vi "Controle_Manip_Main_GUI_WorkingBackup_211222.vi"() -> ()   [LabVIEW 2019]
doc: "VI for micro-photoluminescence setup in GH013 to study the emission properties of single nanoemitters in the visible range.\n\nCoded by Mohamed-Raouf Amara"
uses:
  subVIs/TypeDefs/AcqMode.ctl
  C:/Users/manip/Documents/Controle_Manip_2020/Thorlabs.MotionControl.Controls.dll
  Thorlabs.MotionControl.Controls.dll
  C:/Users/manip/Documents/Controle_Manip_2020/Thorlabs.MotionControl.KCube.SolenoidCLI.dll
  Thorlabs.MotionControl.KCube.SolenoidCLI.dll
  C:/Users/manip/Documents/Controle_Manip_2020/Thorlabs.MotionControl.KCube.PiezoCLI.dll
  Thorlabs.MotionControl.KCube.PiezoCLI.dll
  subVIs/Light Field/lightfield-automation-labview/LightField Automation.lvclass
  C:/Program Files/Thorlabs/Scientific Imaging/DCx Camera Support/Develop/DotNet/uc480DotNet.dll
  Program Files/Thorlabs/Scientific Imaging/DCx Camera Support/Develop/DotNet/uc480DotNet.dll
  subVIs/Light Field/lightfield-automation-labview/VIs/TypeDefs/OpticalPortLocation.ctl
  <vilib>/Analysis/baseanly.llb/Mean (DBL).vi
  subVIs/Globals/InstrumentsOn.vi
  subVIs/Globals/InstrumentReferences.vi
  <vilib>/DAQmx/create/channels.llb/DAQmx Create Channel (AO-Voltage-Basic).vi
  subVIs/Attocubes/ANC350_4.2.4_LV16.llb/ANC350v4sub_setFrequency.vi
  subVIs/Attocubes/ANC350_4.2.4_LV16.llb/ANC350v4sub_setAmplitude.vi
  subVIs/Attocubes/ANC350_4.2.4_LV16.llb/ANC350v4sub_getFrequency.vi
  subVIs/Attocubes/ANC350_4.2.4_LV16.llb/ANC350v4sub_getAmplitude.vi
  subVIs/Newport/Newport ESP301/Newport ESP301.lvlib
  <vilib>/Analysis/NI_AALBase.lvlib
panel:
  out "PuissancesPolar":dbl[](array[numeric])
  out "LLTFDevice error out":errorcluster
  out "LLTFDevice Interface":refnum<k7>
  out "LLTF Error":errorcluster
  out "LLTF Reference":refnum<k7>
  in  "xphyspecLib.IXPhySpec":refnum<k7>
  out "PLE 2D ExcWL&Pow":dbl[][](array[numeric])
  out "PLE ExcWL":dbl[](array[numeric])
  out "PLE Norm Int":dbl[][](array[numeric])
  out "PLE Raw Int":i32[][](array[numeric])
  out "PLE IntegInten":dbl[](array[numeric])
  out "PLE ExcPow":dbl[](array[numeric])
  out "Scan Polar AllParams":refnum<vi>[](array[refnum])
  out "Scan PLE AllParams":refnum<vi>[](array[refnum])
  out "Scan PLE Params":refnum<vi>[](array[refnum])
  out "Scan PLE":T1
  out "ExperimentStopped?":bool
  in  "StopPolar":bool
  in  "PausePolar":bool
  out "Elapsed (s)":dbl
  out "Expected (s)":dbl caption="/"
  in  "Stop fPow":bool
  in  "Pause fPow":bool
  in  "MasterStop":bool
  in  "MasterPause":bool
  out "imagefilename":string
  out "Experiment Name With Date":string
  out "FullComment":string
  out "WrittenDatasetName":string
  out "LastDotNum":dbl min=1.0
  out "output cluster":T2
  out "Params Save":T4
  out "Location cluster":T5
  out "Location Parameters":T6
  out "XYPositions":dbl[][](array[numeric])=[[-0.09999999999999998, -0.3], [-0.09999999999999998, -0.19999999999999996], [-0.3, 0.4], [0.20000000000000007, -0.09999999999999998], [-0.5, -0.5], [0.0, 0.20000000000000007], [0.30000000000000004, 0.30000000000000004], [-0.3, -0.5], [-0.5, 0.10000000000000009], [0.0, 0.4], [0.20000000000000007, 0.10000000000000009], [0.30000000000000004, 0.0], [-0.09999999999999998, -0.4], [-0.4, -0.19999999999999996], [-0.5, -0.19999999999999996], [0.4, 0.4], [-0.5, -0.4], [-0.5, -0.3], [-0.19999999999999996, 0.10000000000000009], [-0.19999999999999996, 0.4], [0.4, -0.5], [0.0, 0.10000000000000009], [-0.19999999999999996, 0.0], [0.10000000000000009, 0.30000000000000004], [-0.3, 0.10000000000000009], [0.10000000000000009, -0.3], [0.20000000000000007, -0.4], [-0.09999999999999998, 0.0], [-0.4, -0.5], [-0.5, 0.0], [-0.3, 0.20000000000000007], [-0.5, 0.20000000000000007], [-0.19999999999999996, 0.20000000000000007], [0.5, 0.4], [-0.4, 0.5], [0.5, 0.0], [0.5, 0.20000000000000007], [0.20000000000000007, -0.19999999999999996], [0.10000000000000009, -0.5], [0.4, 0.30000000000000004], [0.10000000000000009, 0.10000000000000009], [-0.4, 0.10000000000000009], [-0.5, 0.30000000000000004], [0.30000000000000004, -0.19999999999999996], [-0.09999999999999998, -0.5], [0.10000000000000009, -0.4], [0.20000000000000007, 0.5], [-0.3, -0.3], [0.4, 0.5], [0.30000000000000004, 0.5], [0.5, -0.3], [-0.09999999999999998, 0.30000000000000004], [0.10000000000000009, 0.20000000000000007], [0.5, 0.10000000000000009], [0.20000000000000007, 0.20000000000000007], [0.5, -0.5], [0.0, -0.5], [0.10000000000000009, 0.0], [0.10000000000000009, -0.19999999999999996], [-0.3, -0.19999999999999996], [-0.4, -0.09999999999999998], [0.20000000000000007, 0.30000000000000004], [0.20000000000000007, -0.5], [-0.3, 0.5], [0.4, 0.10000000000000009], [-0.3, -0.09999999999999998], [0.30000000000000004, -0.4], [0.30000000000000004, 0.10000000000000009], [0.30000000000000004, -0.3], [-0.4, 0.4], [0.5, -0.4], [-0.19999999999999996, -0.19999999999999996], [0.0, -0.19999999999999996], [0.4, 0.20000000000000007], [0.0, 0.0], [0.30000000000000004, 0.20000000000000007], [-0.09999999999999998, 0.5], [-0.3, -0.4], [0.4, -0.3], [0.0, 0.30000000000000004], [0.30000000000000004, 0.4], [0.0, -0.4], [-0.4, 0.30000000000000004], [0.20000000000000007, 0.4], [-0.5, 0.5], [-0.4, -0.4], [0.30000000000000004, -0.5], [0.10000000000000009, 0.4], [-0.09999999999999998, 0.10000000000000009], [0.10000000000000009, 0.5], [-0.4, -0.3], [0.5, -0.09999999999999998], [-0.5, -0.09999999999999998], [0.0, -0.09999999999999998], [-0.19999999999999996, -0.5], [0.4, 0.0], [0.0, -0.3], [-0.19999999999999996, 0.5], [0.5, -0.19999999999999996], [-0.09999999999999998, 0.20000000000000007], [-0.19999999999999996, -0.09999999999999998], [0.20000000000000007, 0.0], [-0.19999999999999996, 0.30000000000000004], [-0.19999999999999996, -0.3], [-0.5, 0.4], [0.10000000000000009, -0.09999999999999998], [-0.19999999999999996, -0.4], [-0.09999999999999998, 0.4], [0.30000000000000004, -0.09999999999999998], [-0.09999999999999998, -0.09999999999999998], [0.20000000000000007, -0.3], [-0.4, 0.20000000000000007], [0.4, -0.4], [-0.3, 0.30000000000000004], [0.5, 0.5], [0.4, -0.19999999999999996], [-0.3, 0.0], [0.0, 0.5], [0.5, 0.30000000000000004], [0.4, -0.09999999999999998], [-0.4, 0.0]]
  in  "DotNum":dbl=1.0 min=1.0
  out "Array fPow Pow":dbl[](array[numeric])
  out "Array fPow":i32[][](array[numeric])
  out "Scan XY Map Exp Params SubVI":T7
  out "Scan XY Map Exp Params SubVI Mod":T8
  out "Scan XY Map References":T9
  in  "Display Mode":u16(ring) items=["Sum", "Max", "Sum/s", "Max/s", "Efficiency"]
  out "BackgroundSpec":dbl[](array[numeric])
  out "Cnts":dbl caption="cnts" format="%_3p"
  out "XYPos Indices":i32[][](array[numeric])
  out "best fit parameters":dbl[](array[numeric])
  out "Image":dbl[][][](array[numeric])
  out "Data PL Custom Diode Spectrum":dbl[](array[numeric])
  out "Out Position [µm | m°]":dbl
  in  "Reset origins":bool
  in  "Delay Line Position (mm)":dbl caption="Delay line position (mm)"
  out "PD Data 2D 2":dbl[][](array[numeric])
  out "PH_Settings_Params":T10={"SyncDiv"=1, "DeviceIndex"=0, "CFD0 level"=50, "CFD0 zero X"=10, "CFD1 level"=50, "CFD1 zero X"=10, "Range No."=0, "StopOnOverflow"=FALSE, "AcqTime (ms)"=0.0} {"Range No." min=0 max=5 step=1; "CFD1 zero X" min=0 max=40 step=1; "CFD1 level" min=0 max=400 step=1; "CFD0 zero X" min=-1300 max=400 step=10; "CFD0 level" min=-1300 max=400 step=10; "SyncDiv" min=1 max=8 step=1}
  out "PH_Init_Data":T11
  out "NewVal":bool
  out "Scan XY Map Handles":T12
  out "Constrast Handles":T13
  out "Contrast References":T14
  in  "Acquire MyPol":bool
  out "Polar Params SubVIv2":T15
  out "Test Handles Polar":T16
  out "Scan Polarisation References":T17
  in  "Att Stop Wobble":bool
  out "Scan Main Progess Bar":u8(slide) scale=0.0..100.0
  out "XYMap Data":i32[][](array[numeric])
  out "PD Data":dbl[](array[numeric])
  out "DDE":refnum<visa-resource-name> caption="resource name"
  in  "Acquire Spectrum Custom":bool
  in  "Stop Spectrum Customm":bool
  out "Scan Spectrum Cust Exp Params":T18
  in  "Experimental parameters tab":T19(tab)
  in  "Save PLE":bool
  in  "Acquire PLE":bool
  in  "PLE Step (nm)":dbl=0.1 caption="Step (nm)" min=0.01 max=100.0 step=0.05
  in  "PLE End (nm)":dbl=500.0 caption="End (nm)" min=300.0 max=1200.0
  in  "PLE Start (nm)":dbl=400.0 caption="Start (nm)" min=300.0 max=1200.0
  out "Background taken?":bool
  in  "Save Custom Diode Spectrum":bool
  in  "Acquire Custom Diode Spectrum":bool
  in  "N Step Power  Diode Current (A)":i32=20 caption="N Steps" min=2 step=1
  in  "End Power  Diod Current (A)":dbl=0.04 caption="End (A)" min=0.02 max=0.0605
  in  "Start Power Diod Current (A)":dbl=0.02 caption="Start (A)" min=0.02 max=0.0605
  in  "Mono2 Wavelength (nm)":dbl=300.0 caption="Wavelength (nm)" min=300.0 max=1000.0 step=0.1
  in  "Mono2 Motor Pos":dbl caption="Motor Pos"
  out "Mono2 On":bool caption="Motor On?"
  in  "CCD ROI":T20(ring) caption="ROI"
  in  "Spectrum Step Wavelength (nm)":dbl=0.25 caption="Step (nm)" min=-100.0 max=100.0 step=0.05
  in  "Spectrum End Wavelength (nm)":dbl=350.0 caption="End (nm)" min=350.0 max=900.0
  in  "Spectrum Start Wavelength (nm)":dbl=350.0 caption="Start (nm)" min=350.0 max=900.0
  in  "Accumulations":dbl=1.0 caption="Acc." min=1.0 step=1.0
  in  "Background substract":enum16{"None", "Shutter"}(ring) caption="Bkg substract"
  in  "Exit mirror":u16(ring)=4 caption="ExitPort :" items=["CCD"=4, "APD"=5]
  in  "Center Wavelength (nm)":dbl=448.9 caption="Center WL :" min=0.0 max=2000.0 step=0.01
  in  "Exposure Time (ms)":dbl=500.0 caption="Exposure :" min=1.0 max=360000.0 step=1.0
  in  "Grating":string(combo)="[h-vis,2400][0][0]" caption="Grating :"
  in  "Spectrum Custom Mode":u16(ring)=1 caption="Detector" items=["PD 1", "APD 1", "APD 2", "APD 1+2", "PD 2"]
  in  "Stop Spectrum Custom":bool
  in  "Save fPow":bool
  in  "Acquire fPow":bool
  in  "HR mode":u16(ring)=1 caption="Which HR?" items=["Excitation"=2, "Detection"=1]
  out "PLE # Pts":dbl=1001.0
  in  "Add location":bool
  in  "Acquire XY Map":bool
  in  "Pause XY Map":bool
  in  "Stop XY Map":bool
  out "Scan X Readout (V)":dbl caption="X Readout" min=-10.0 max=10.0 format="%#.3g"
  out "Scan Y Readout (V)":dbl caption="Y Readout" min=-10.0 max=10.0 format="%#.3g"
  in  "Scan Y Tot. Length":dbl=6.0 caption="Y Length" min=0.0 max=20.0 step=0.5
  in  "Scan X Tot. Length (V)":dbl=6.0 caption="X Length (V)" min=0.0 max=20.0 step=0.5
  out "Scan Y Num. Pts":dbl=121.0 caption="Y # Pts"
  out "Scan X Num. Pts":dbl=121.0 caption="X # Pts"
  in  "Scan Y Res. (V)":dbl=0.05 caption="Res. Y (V)" min=0.0 max=5.0 step=0.05
  in  "Scan X Res. (V)":dbl=0.05 caption="Res. X (V)" min=0.0 max=5.0 step=0.05
  in  "Scan Y Center (V)":dbl caption="Y Center (V)"
  in  "Scan X Center (V)":dbl caption="X Center (V)"
  in  "FSM Home":bool
  in  "FSM Right":bool
  in  "FSM Left":bool
  in  "FSM Down":bool
  in  "FSM Up":bool
  in  "FSM X Axis Pos":dbl caption="Target X" min=-10.0 max=10.0 format="%#.3g"
  in  "FSM Y Axis Pos":dbl caption="Target Y" min=-10.0 max=10.0 format="%#.3f"
  in  "FSM Axis Step":dbl=0.1 caption="Step"
  in  "Save XY Map":bool
  in  "Scanning Mode":T21(ring) caption="Mode"
  in  "Scan Fast Axis":enum16{"Y", "X"}(ring)=enum."X" caption="Fast Axis"
  in  "ZDummyCluster MHILS 3":cluster{"Stop":bool}
  in  "Map Marker X Pos":i8=1 min=1 max=50 step=1
  in  "Map Marker Y Pos":i8=1 min=1 max=50
  in  "Pol in path?":bool
  out "RotStage Det Angle Readout (°)":dbl=2.0 caption="Readout (°)" min=-3600.0 max=125.0 format="%#_4g"
  out "RotStage Exc Angle Readout (°)":dbl=2.0 caption="Readout (°)" min=-360.0 max=360.0 format="%#_4g"
  in  "Acquire Polarisation":bool
  in  "RotStage Det Angle Step (°)":dbl=10.0 caption="Step (°)"
  in  "RotStage Exc Angle Step (°)":dbl=10.0 caption="Step (°)"
  in  "RotStage Det Jog Forward":bool
  in  "RotStage Exc Jog Forward":bool
  in  "RotStage Det Jog Backward":bool
  in  "RotStage Det Home":bool caption="Home"
  in  "RotStage Exc Home":bool caption="Home"
  in  "RotStage Det Angle (°)":dbl caption="Target (°)" min=0.0 max=3600.0 format="%#_4g"
  in  "RotStage Exc Angle (°)":dbl caption="Target (°)" min=0.0 max=3600.0 format="%#_4g"
  in  "RotStage Exc Jog Backward":bool
  in  "Polar Start Angle (°)":dbl caption="Start angle (°)" min=-360.0 max=360.0 step=10.0
  in  "Polar End Angle (°)":dbl=360.0 caption="End Angle (°)" min=0.0 max=360.0 step=10.0
  in  "Polar Step Angle (°)":dbl=10.0 caption="Step Angle (°)" min=0.01 max=360.0
  in  "Polar mode":u16(ring)=3 caption="Rotate HWP" items=["Excitation"=3, "Detection"=2]
  in  "Save Polarisation":bool
  in  "RotStage Det Velocity (°/s)":dbl=2.0 caption="Velocity (°/s)" min=0.0 max=20.0 step=1.0
  in  "RotStage Exc Velocity (°/s)":dbl=2.0 caption="Velocity (°/s)" min=0.0 max=20.0 step=1.0
  in  "Motor RotStage Exc On?":bool
  in  "Motor RotStage Det On?":bool
  in  "ZDummyCluster MHILS 2":cluster{"Stop":bool}
  out "Scan Michelson Progess Bar":u8(slide) scale=0.0..100.0
  in  "Stop Michelson":bool
  in  "Pause Michelson":bool
  in  "Save Michelson":bool
  in  "Acquire Michelson":bool
  in  "Stop Contrast":bool
  in  "Pause Contrast":bool
  in  "Save Contrast":bool
  in  "Newport PZA12 Stage Position (usteps)":dbl caption="Target (ustp)" min=-8.0 max=392.0
  in  "LinTFine Motor On?":bool caption="Motor on?"
  in  "Acquire Contrast":bool
  in  "LinTFines Step Pos (usteps)":dbl=1.0 caption="Step pos (usteps)" min=1.0 max=100.0 step=1.0
  in  "LinTFine End Pos (usteps)":dbl=10.0 caption="End pos (usteps)" min=-1000000.0 max=1000000.0 step=1.0
  in  "LinTFine Start Pos (usteps)":dbl caption="Start pos (usteps)" min=-1000000.0 max=1000000.0 step=1.0
  in  "PZC Speed (usteps/s)":u16(ring) caption="Velocity (ustp/s)" items=["0", "3.2", "16", "80", "400", "2000", "10000", "48000"]
  in  "PZC Jog Forward":bool
  in  "PZC Jog Backward":bool
  in  "PZC Home":bool caption="Home"
  out "PZC Position Readout (usteps)":dbl caption="Readout (ustp)" min=-8.0 max=392.0
  out "Newport Linear Translation Stage Position Readout (mm)":dbl caption="Readout (mm)" min=-8.0 max=392.0 format="%#_7g"
  in  "Newport Linear Translation Stage Step (mm)":dbl=5.0 caption="Step (mm)"
  in  "Newport Linear Translation Stage Position (mm)":dbl caption="Target (mm)" min=-125.0 max=125.0
  out "Scan Linear Stage Progess Bar":u8(slide) scale=0.0..100.0
  in  "Newport Linear Translation Stage Home":bool caption="Home"
  in  "Newport Linear Translation Stage Jog Forward":bool
  in  "Newport Linear Translation Stage Jog Backward":bool
  in  "Newport Linear Translation Stage Velocity (mm/s)":dbl=1.0 caption="Velocity (mm/s)" min=0.0 max=100.0 step=1.0
  in  "LinT Step Pos (mm)":dbl=10.0 caption="Step pos (mm)" min=-50.0 max=50.0 step=0.001
  in  "LinT End pos (mm)":dbl caption="End pos (mm)" min=-250.0 max=0.0 step=10.0
  in  "LinT Start Pos (mm)":dbl caption="Start pos (mm)" min=-5.0 max=200.0 step=10.0
  in  "Motor LinT On?":bool
  out "Michelson Elapsed (s)":dbl format="%#_4g"
  out "Michelson Expected (s)":dbl caption="/" format="%#_4g"
  in  "ZDummyCluster MHILS":cluster{"Stop":bool}
  in  "Tab Objective Sample":T22(tab)
  in  "KCubePiezoControl X":refnum<k24>(container) caption="Lateral"
  in  "KCubePiezoControl Y":refnum<k24>(container) caption="Vertical"
  in  "KCubePiezoControl Z":refnum<k24>(container) caption="Focus"
  out "GetOutputVoltage":dbl
  out "IsSetOutputVoltageActive":bool
  in  "Att Wobble Get Pos 2":bool
  in  "Att Wobble Get Pos 1":bool
  in  "Att Mode":enum16{"Single Step", "Continuous", "Automatic"}(ring)
  in  "Voltage Output?":bool caption="Vout?"
  in  "Att AutoStep":dbl caption="Auto Step" min=-3000.0 max=3000.0
  in  "Att DCLvl":dbl caption="DC Level" min=0.0 max=70.0
  in  "Att Freq":dbl=1000.0 caption="Frequency (Hz)" min=0.0 max=2000.0
  in  "Att Amp":dbl=30.0 caption="Amplitude" min=0.0 max=70.0
  in  "Att Stop Motion":bool
  in  "Att Up":bool
  in  "Att Down":bool
  in  "Att Left":bool
  in  "Att Right":bool
  in  "Att Backward":bool
  in  "Att Forward":bool
  in  "Att Pos X":dbl min=-500.0 max=3500.0 format="%#_7g"
  in  "Att Pos Y":dbl min=-500.0 max=3500.0 format="%#_7g"
  in  "Att Pos Z":dbl min=-500.0 max=3500.0 format="%#_7g"
  in  "Att Read Pos":bool
  in  "ANC Axis":u8(ring) items=["1", "2", "3"]
  in  "Att Stop Target Wait":bool
  in  "Att Track Target":bool
  in  "Att Wobble":bool
  in  "Att Wobble Start":dbl caption="Start"
  in  "Att Wobble End":dbl caption="End"
  in  "Att Wobble Stop2":bool
  in  "KCubeSolenoidControl":refnum<k24>(container)
  in  "Shutter Mode":i32(ring)=1 items=["Manual"=1, "SingleToggle"=2, "AutoToggle"=3, "Triggered"=4]
  out "CCD 1D Spectrum XY Map":dbl[][](graph)
  out "Params XY Map SubVI":T23
  out "Att DeviceHandle":u64
  in  "Thorcam":bool
  out "Scan Translation Exp Params":T24
  in  "Fast Acq Continuous":bool
  in  "Fast Acq":bool
  out "Shutter Ctrls":u16(ring)
  out "Laser on?":bool
  out "Excitation Power (uW)":dbl=0.2 caption="P    =" format="%#_3p"
  in  "Acq Time (ms)":dbl=250.0 caption="T" min=1.0 max=360000.0 step=50.0
  in  "Auto< ?":bool
  in  "Acq Mode":T3=enum."Spectrum" caption="Mode :"
  in  "Comment":string
  out "Log file":string caption="Status"
  in  "Experiment Name":string="NewB"
  in  "Experiment Graph Controls":T25(tab)
  in  "Fit?":bool
  out "Duration":dbl caption="s"
  in  "Acquire N: N":dbl=10.0 caption="N"
  in  "Acquire Time Trace":bool caption="Acquire N"
  in  "CCD 1D Spectrum Main  Cursor2WL 2 Mono 2":bool caption="CCD 1D Spectrum Main  Cursor2WL"
  in  "CCD 1D Spectrum Main  Cursor2WL 1 Mono 2":bool caption="CCD 1D Spectrum Main  Cursor2WL"
  in  "CCD 1D Spectrum Main  Cursor2WL 2 Mono 1":bool caption="CCD 1D Spectrum Main  Cursor2WL"
  in  "CCD 1D Spectrum Main  Cursor2WL 1 Mono 1":bool caption="CCD 1D Spectrum Main  Cursor2WL"
  out "CCD 1D Spectrum Main Cursor 1 nm":dbl caption="nm"
  out "CCD 1D Spectrum Main Cursor 2 nm":dbl caption="nm"
  in  "Full scale":bool
  in  "Acquire Spectrum":bool
  out "CCD 2D Image Main":dbl[][](graph)
  in  "Save Spectrum N":bool
  in  "Save Spectrum":bool
  out "CCD 1D Spectrum Main":cluster{dbl[], dbl[]}(graph) caption="Main spectrum"
  out "CCD 1D Spectrum Main Energy Scale":cluster{dbl[], dbl[]}(graph)
  out "CCD 1D Spectrum Main Cursor":dbl caption="eV" format="%#_6p"
  out "CCD 1D Spectrum Main Cursor 2":dbl caption="eV" format="%#_6p"
  out "CCD 1D Spectrum Main deltaE":dbl caption="eV" format="%#_3p"
  out "CCD 1D Spectrum Main deltanm":dbl caption="m" format="%#_3p"
  in  "Scan FSM Set as Center":bool
  in  "Scan FSM Go to Cursor":bool
  out "XY Intensity Map":dbl[][](graph)
  out "CCD 2D Image XY Map":dbl[][](graph)
  out "CCD 1D Spectrum XY Map":cluster{dbl[], dbl[]}(graph) caption="Current spectrum in XY Map"
  out "CCD 1D XY Map Spectrum Main Energy Scale":cluster{dbl[], dbl[]}(graph)
  in  "NewDot":bool caption="NewDot?"
  out "ExportMapPosition?":bool caption="Export NC Pos in Map Image?"
  out "Polarisation 2D Image":dbl[][](graph) caption="Polarisation Image"
  out "Polarisation 1D Spectrum":cluster{dbl[], dbl[]}(graph) caption="39.6°"
  out "Polarisation 1D Spectrum Energy Scale":cluster{dbl[], dbl[]}(graph)
  out "Contrast":dbl format="%#_3g"
  out "Contrast Oscillations":cluster{dbl[], dbl[]}(graph)
  out "Contrast 1D Spectrum":cluster{dbl[], dbl[]}(graph) caption="52924"
  in  "Cursor controls":bool
  out "Contrast 1D Spectrum from Cursors":cluster{dbl[], dbl[]}(graph) caption="2708"
  in  "Spectrum Custom Continuous Mode":u16(ring)=1 caption="Detector(s)" items=["PD", "APD 1", "APD 2", "APD 1+2"]
  in  "Stop PD":bool
  in  "Acquire PD":bool
  out "PD 1D Spectrum":dbl[][](graph) caption="(A)PDs readout"
  in  "PH_SyncDiv":enum16{"1", "2", "4", "8"}(ring) caption="SyncDiv"
  in  "PH_CFD0 level":i32=50 caption="CFD0" min=0 max=100
  in  "PH_CFD0 zero X":i32=10 caption="CFD0 ZeroX"
  in  "PH_CFD1 level":i32=50 caption="CFD1" min=0 max=100
  in  "PH_CFD1 zero X":i32=10 caption="CFD1 Zero X"
  in  "PH_Range No.":i32 caption="Range No."
  out "PLE Integrated emission efficiency":dbl[](graph)
  out "PLE Normalised Intensity":dbl[][](graph)
  out "PLE Laser Excitation Power":dbl[](graph)
  out "PLE Raw Intensity":i32[][](graph)
  in  "V2um":dbl=10.0
  in  "Conv/Energy (eV)":dbl caption="Energy :" format="%#_6p"
  in  "Conv/Wavelength (nm)":dbl caption="Wavelength :"
  in  "Conv/Wavenumber (m-1)":dbl caption="Wavenumber :"
  in  "Conv/Time (s)":dbl caption="Time :" format="%#_6p"
  in  "Doc FSM":bool
  in  "Doc ESP 300":bool
  in  "Doc Photodiode":bool
  in  "Doc PicoHarp":bool
  in  "Doc LightField":bool
  in  "Doc Attocubes":bool
  in  "Doc NanoMax":bool
  in  "Doc PZC200":bool
  in  "Doc Shutter":bool
  in  "Doc ESP 301":bool
  in  "Doc LLTF":bool
  in  "Doc Cryostat":bool
  out "Connected":bool
  in  "Connect":bool
  out "CurrentWL":dbl
  in  "ChangeSample":bool
  in  "SampleGoal":string
  in  "Write to Markdown?":bool=TRUE
  in  "Synthesis/Solvent":string(combo)="tol"
  in  "Synthesis/Polymer":string(combo)="PS"
  in  "Synthesis/DilutionPolyRatio":dbl=1.5
  in  "SampleOf":string(combo)="CsPbBr3 NCs"
  in  "Synthesis/Dilution":dbl=8000.0
  in  "Synthesis/Name":string(combo)="NewB2"
  in  "Mono2 Velocity":dbl caption="Veloc." min=0.0 max=20.0 step=0.01
  out "ANC connected":bool
  in  "PicoHarp On?":bool
  in  "Cryostation On?":bool
  in  "Attocubes On?":bool
  in  "PZC200 On?":bool
  in  "KCube Shutter On?":bool
  in  "KCubes Piezo On?":bool
  in  "LightField On?":bool
  in  "PM16-120 On?":bool
  in  "ESP 300 On?":bool
  in  "ESP 301 On?":bool
  in  "FSM 300 On?":bool
  out "Cryo User Stability":dbl=450.0 caption="Stability" min=400.0 max=1100.0 step=1.0 format="%#_6p"
  out "Cryo User Temp":dbl=450.0 caption="User" min=400.0 max=1100.0 step=1.0
  out "Cryo Sample Stability":dbl=450.0 caption="Stability" min=400.0 max=1100.0 step=1.0 format="%#_6p"
  out "Cryo Sample Temp":dbl=450.0 caption="Sample" min=400.0 max=1100.0 step=1.0
  out "Cryo Platform Stability":dbl=450.0 caption="Stability" min=400.0 max=1100.0 step=1.0 format="%#_6p"
  out "Cryo Platform Temp":dbl=450.0 caption="Platform" min=400.0 max=1100.0 step=1.0
  in  "PZC200 COM Port":dbl=6.0 caption="COM Port"
  in  "Laser Diode Current Set":dbl(slide)=0.02 caption="Power" min=0.02 max=0.115 scale=0.02..0.0605 scale format="%#_3g"
  in  "Laser on? Control":bool
  in  "Diode Driver COM":refnum<visa-resource-name>="USB0::0x1313::0x804F::M00549740::INSTR"
  in  "Laser Comm On?":bool
  out "ESP300 COM Port":refnum<visa-resource-name>="COM4" caption="COM Port"
  in  "Excitation Wavelength (nm)":dbl=450.0 caption="Exc WL (nm)" min=400.0 max=600.0 step=1.0
  out "Photodiode Status":bool caption="Status"
  in  "ESP 301 COM Port":refnum<visa-resource-name>="ASRL8::INSTR" caption="COM Port"
  in  "FSM Y Axis":tag="cDAQ2Mod1/ao1"
  in  "FSM X Axis":tag="cDAQ2Mod1/ao2"
  in  "Slit Width (mm)":dbl caption="Slit (mm)" min=0.0 max=5.0 step=0.01
  out "Initialise all devices?":bool caption="OK"
  in  "TEC Output":bool
  out "TEC Temperature":dbl caption="TEC Temp" format="%#_4f"
  out "Laser Safety":u16(ring)
  in  "LF Visible":bool=TRUE caption="LF Visible ?"
  out "PZC200 Instrument Channel":string="RS232/10" caption="PZC200 Port"
  out "Cryostation ID":refnum<k5>
  out "Serial Number":string caption="Serial"
  out "FSM X Task":refnum<k21>
  out "FSM Y Task":refnum<k21>
  in  "Cryostat":enum16{"Montana", "Oxford"}(ring) caption="Cryo :"
  out "CCD T° :":dbl
  in  "Synthesis/InjTemp":dbl=180.0
  in  "Sample first cooldown":timestamp=timestamp(3709040400 s since 1904-01-01) format="%<%x %.3X>T"
  in  "LLTF On?":bool
  out "LLTF Detected?":bool
  out "CurrentAngle":dbl
  out "Device moved":bool
  in  "FocalShift (V KCube)":dbl
  out "PZAPos&Pow":dbl[][](array[numeric])
  out "PZC Error":errorcluster
  in  "ESP 301 Error":errorcluster
  out "KCubeSolenoidControl Reference":refnum<k24>
  out "KCube Shutter Device Reference":refnum<k24>
  out "KCubePiezoDevice Z Reference":refnum<k24>
  out "KCubePiezoControl Z Reference":refnum<k24>
  out "KCubePiezoControl Y Reference":refnum<k24>
  out "KCubePiezoDevice Y Reference":refnum<k24>
  out "KCubePiezoDevice X Reference":refnum<k24>
  out "KCubePiezoControl X Reference":refnum<k24>
  out "Wavelength calibration":dbl[](array[numeric])
  out "Photodiode handle out":refnum<visa-resource-name> caption="instrument handle out"
  out "Photodiode error out":errorcluster caption="error out" {"code" format="%.0x"}
  out "LightField Automation error out":errorcluster
  out "Scan Polar Params":refnum<vi>[](array[refnum])
  out "Angles":dbl[](array[numeric])
  out "Scan XY Map Params":refnum<vi>[](array[refnum])
  out "Thorcam Error":errorcluster caption="Error Out"
  out "Data":T26(array[cluster])
  in  "ESP300 Error":errorcluster
  out "ThorCam Reference":refnum<k24>
  out "LightField Automation out":refnum<class "LightField Automation.lvclass">
  out "Response":string
  out "PZA12 Positions":dbl[](array[numeric])
  out "Contrast Array Out":dbl[][](array[numeric])
  out "Michelson Array Out":dbl[][][](array[numeric])
  out "Pol 2D Array Out":dbl[][](array[numeric])
  out "PZC&Pow3D":dbl[][][](array[numeric])
  out "Scan Translation Params":T27
  out "Scan Contrast Ctrls":refnum<vi>[](array[refnum])
  out "ESP Pos":dbl[](array[numeric])
  out "ourDLL":path
  out "Diode Driver Error out":errorcluster
  out "Diode Driver Error":errorcluster caption="error in (no error)" {"code" format="%.0x"}
  out "Scan Translation Coarse Ctrls":refnum<vi>[](array[refnum])
  out "Scan Spectrum Cust Params":refnum<vi>[](array[refnum])
  out "Position (units)":dbl format="%.6g"
  out "Att Error":errorcluster
  in  "Stop Everything & Quit?":bool
  in  "Excitation Source":enum16{"P", "CW", "SK"}(ring)=enum."CW" caption="Laser"
  in  "Temperature (K)":dbl=5.0 caption="T ="
  # "P"
  # "K"
  # "NC"
  # "acq"
  # "s"
  # "Possibly add a slit size option to determine the resolution"
  # "add functionnality spectrum with APD 1 or APD 2"
  # "Controls"
  # "Scans"
  # "Scan detection wavelength"
  # "SpectraPro"
  # "Vary excitation power"
  # "better use\nHWP"
  # "f(Power)"
  # "Pixis CCD"
  # "Vary excitation wavelength PLE with filtered SuperK"
  # "JY HR320"
  # "nm"
  # "ms"
  # "Controls"
  # "Scans"
  # "+"
  # "Scanning sample area with marker:"
  # "Fast steering mirror"
  # "Scan laser spot with mirror and acquire spectra"
  # "Controls"
  # "Scans"
  # "in path?"
  # "Excitation"
  # "Rotate half-wave plate and acquire spectra"
  # "Detection"
  # "Controls"
  # "Scans"
  # "Coarse translation stage"
  # "Michelson"
  # "Contrast"
  # "Fine translation stage"
  # "Y"
  # "X"
  # "Z"
  # "Scans"
  # "Y"
  # "X"
  # "Wobble"
  # "Z"
  # "exc"
  # "W"
  # "ms"
  # "Mono 1"
  # "Mono 2"
  # "--|--"
  # "Acquisition"
  # "CenterWL"
  # "l   ="
  # "E  ="
  # "DE ="
  # "1"
  # "1"
  # "--|--"
  # "Dl ="
  # "f(time)"
  # "CenterWL"
  # "l   ="
  # "E   ="
  # "2"
  # "2"
  # "and increment NC number"
  # "Current spectrum from polar"
  # "Current spectrum from constrast"
  # "CFD"
  # "Zero Cross"
  # "Sync/CH0"
  # "CFD"
  # "CH1"
  # "Zero Cross"
  # "Absolute conversions"
  # "change one value manually and the others will update accordingly"
  # "Detection efficiency"
  # "For the steering mirror, in the current configuration 1 V equals to                um."
  # "eV"
  # "nm"
  # "-1"
  # "cm"
  # "s"
  # "Thorlabs Laser Diode Driver CLD1010"
  # "min"
  # "max"
  # "Newport FSM-300-01"
  # "Newport ESP 301"
  # "Laser Line Tunable Filter"
  # "Axis 2: Det"
  # "Axis 3: Exc"
  # "Axis 1"
  # "Montana Cryostation s50"
  # "Newport PZC200"
  # "Thorlabs Shutter SH05"
  # "Thorlabs NanoMax + 3 Axis Piezos"
  # "Attocube ANC350 - 2 ANPx51 & 1 ANPz51"
  # "Synthesis and sample details"
  # "Inside the cryostat, there is a sample of"
  # "Newport ESP 300"
  # "The sample currently inside the cryostat is from the                                 synthesis made"
  # "with an injection temperature of          °C.  The sample was prepared by dispersing"
  # "a solution diluted                     times in a          % solution of                               in                        ."
  # "The sample was prepared on"
  # "PicoHarp 300"
  # "Thorlabs PM16-120"
  # "Princeton HRS-500 + Pixis"
  # "The sample is inside the cryostat in order to:"
  # "°C"
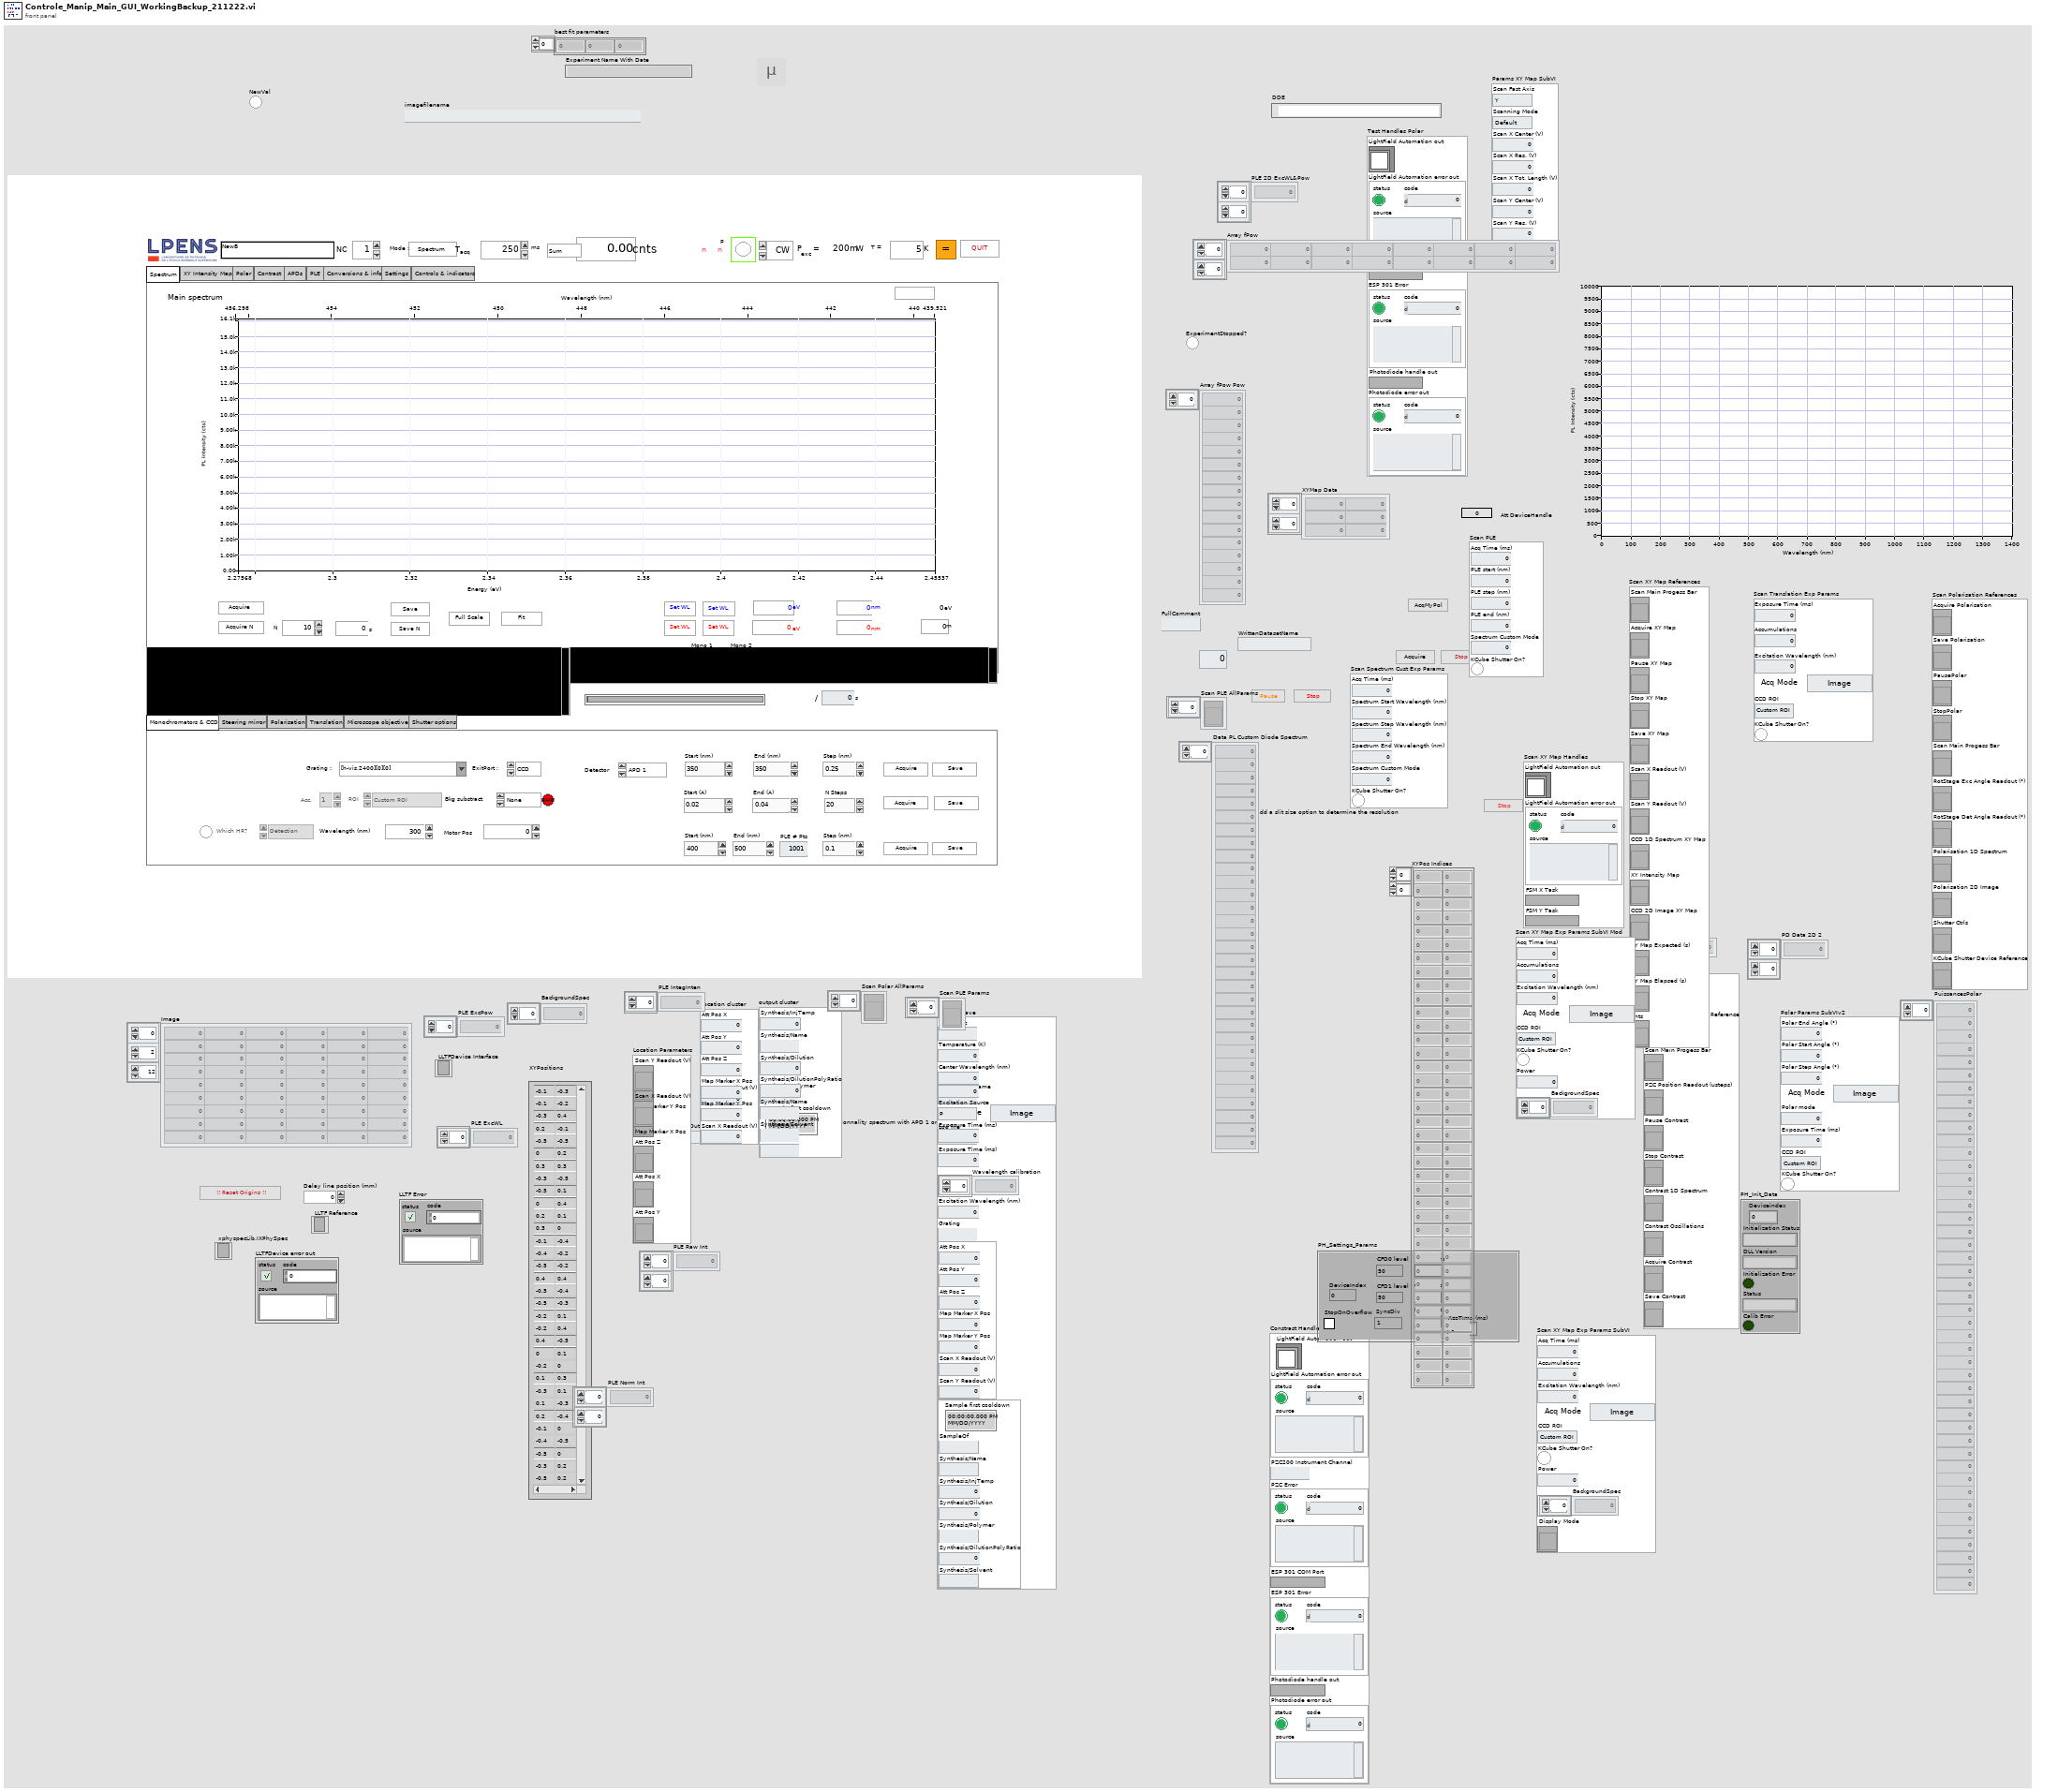
[diagram p1: front panel]
types:
  T1 = cluster{"Acq Time (ms)":dbl, "PLE start (nm)":dbl, "PLE step (nm)":dbl, "PLE end (nm)":dbl, "Spectrum Custom Mode":u16, "KCube Shutter On?":bool}
  T2 = cluster{"Synthesis/InjTemp":dbl, "Synthesis/Name":string, "Synthesis/Dilution":dbl, "Synthesis/DilutionPolyRatio":dbl, "Synthesis/Name":string, "Synthesis/Solvent":string, "Synthesis/Polymer":string, "Sample first cooldown":timestamp, "SampleOf":string}
  T3 = typedef "AcqMode.ctl" = enum16{"Image", "Spectrum", "APD 1", "APD 2", "APD 1+2"}
  T4 = cluster{"Comment":string, "Temperature (K)":dbl, "Center Wavelength (nm)":dbl, "Numeric":dbl, "Excitation Source":enum16{"P", "CW", "SK"}, "Exposure Time (ms)":dbl, "Experiment Name":string, "Acq Mode":T3, "Log file":string, "Exposure Time (ms)":dbl, "Wavelength calibration":dbl[], "Excitation Wavelength (nm)":dbl, "Grating":string, "Cluster":cluster{"Att Pos X":dbl, "Att Pos Y":dbl, "Att Pos Z":dbl, "Map Marker X Pos":i8, "Map Marker Y Pos":i8, "Scan X Readout (V)":dbl, "Scan Y Readout (V)":dbl}, "Cluster":cluster{"Sample first cooldown":timestamp, "SampleOf":string, "Synthesis/Name":string, "Synthesis/InjTemp":dbl, "Synthesis/Dilution":dbl, "Synthesis/Polymer":string, "Synthesis/DilutionPolyRatio":dbl, "Synthesis/Solvent":string}}
  T5 = cluster{"Att Pos X":dbl, "Att Pos Y":dbl, "Att Pos Z":dbl, "Map Marker X Pos":i8, "Map Marker Y Pos":i8, "Scan X Readout (V)":dbl, "Scan Y Readout (V)":dbl}
  T6 = cluster{"Scan Y Readout (V)":refnum<vi>, "Scan X Readout (V)":refnum<vi>, "Map Marker X Pos":refnum<vi>, "Map Marker Y Pos":refnum<vi>, "Att Pos Z":refnum<vi>, "Att Pos X":refnum<vi>, "Att Pos Y":refnum<vi>}
  T7 = cluster{"Acq Time (ms)":dbl, "Accumulations":dbl, "Excitation Wavelength (nm)":dbl, "Acq Mode":T3, "CCD ROI":enum16{"Custom ROI", "Full sensor", "Binned full sensor"}, "KCube Shutter On?":bool, "Power":dbl, "BackgroundSpec":dbl[], "Display Mode":refnum<vi>}
  T8 = cluster{"Acq Time (ms)":dbl, "Accumulations":dbl, "Excitation Wavelength (nm)":dbl, "Acq Mode":T3, "CCD ROI":enum16{"Custom ROI", "Full sensor", "Binned full sensor"}, "KCube Shutter On?":bool, "Power":dbl, "BackgroundSpec":dbl[]}
  T9 = cluster{"Scan Main Progess Bar":refnum<vi>, "Acquire XY Map":refnum<vi>, "Pause XY Map":refnum<vi>, "Stop XY Map":refnum<vi>, "Save XY Map":refnum<vi>, "Scan X Readout (V)":refnum<vi>, "Scan Y Readout (V)":refnum<vi>, "CCD 1D Spectrum XY Map":refnum<vi>, "XY Intensity Map":refnum<vi>, "CCD 2D Image XY Map":refnum<vi>, "XY Map Expected (s)":refnum<vi>, "XY Map Elapsed (s)":refnum<vi>, "Cnts":refnum<vi>}
  T10 = cluster{"SyncDiv":i32, "DeviceIndex":i32, "CFD0 level":i32, "CFD0 zero X":i32, "CFD1 level":i32, "CFD1 zero X":i32, "Range No.":i32, "StopOnOverflow":bool, "AcqTime (ms)":dbl}
  T11 = cluster{"Deviceindex":i32, "Initialization Status":string, "DLL Version":string, "Initialization Error":bool, "Status":string, "Calib Error":bool}
  T12 = cluster{"LightField Automation out":refnum<class "LightField Automation.lvclass">, "LightField Automation error out":errorcluster, "FSM X Task":refnum<k21>, "FSM Y Task":refnum<k21>}
  T13 = cluster{"LightField Automation out":refnum<class "LightField Automation.lvclass">, "LightField Automation error out":errorcluster, "PZC200 Instrument Channel":string, "PZC Error":errorcluster, "ESP 301 COM Port":refnum<visa-resource-name>, "ESP 301 Error":errorcluster, "Photodiode handle out":refnum<visa-resource-name>, "Photodiode error out":errorcluster}
  T14 = cluster{"Shutter Ctrls":refnum<vi>, "KCube Shutter Device Reference":refnum<vi>, "Scan Main Progess Bar":refnum<vi>, "PZC Position Readout (usteps)":refnum<vi>, "Pause Contrast":refnum<vi>, "Stop Contrast":refnum<vi>, "Contrast 1D Spectrum":refnum<vi>, "Contrast Oscillations":refnum<vi>, "Acquire Contrast":refnum<vi>, "Save Contrast":refnum<vi>}
  T15 = cluster{"Polar End Angle (°)":dbl, "Polar Start Angle (°)":dbl, "Polar Step Angle (°)":dbl, "Acq Mode":T3, "Polar mode":u16, "Exposure Time (ms)":dbl, "CCD ROI":enum16{"Custom ROI", "Full sensor", "Binned full sensor"}, "KCube Shutter On?":bool}
  T16 = cluster{"LightField Automation out":refnum<class "LightField Automation.lvclass">, "LightField Automation error out":errorcluster, "ESP 301 COM Port":refnum<visa-resource-name>, "ESP 301 Error":errorcluster, "Photodiode handle out":refnum<visa-resource-name>, "Photodiode error out":errorcluster}
  T17 = cluster{"Acquire Polarisation":refnum<vi>, "Save Polarisation":refnum<vi>, "PausePolar":refnum<vi>, "StopPolar":refnum<vi>, "Scan Main Progess Bar":refnum<vi>, "RotStage Exc Angle Readout (°)":refnum<vi>, "RotStage Det Angle Readout (°)":refnum<vi>, "Polarisation 1D Spectrum":refnum<vi>, "Polarisation 2D Image":refnum<vi>, "Shutter Ctrls":refnum<vi>, "KCube Shutter Device Reference":refnum<vi>}
  T18 = cluster{"Acq Time (ms)":dbl, "Spectrum Start Wavelength (nm)":dbl, "Spectrum Step Wavelength (nm)":dbl, "Spectrum End Wavelength (nm)":dbl, "Spectrum Custom Mode":u16, "KCube Shutter On?":bool}
  T19 = enum32{"Monochromators & CCD", "Steering mirror", "Polarisation", "Translation", "Microscope objective", "Shutter options"}
  T20 = enum16{"Custom ROI", "Full sensor", "Binned full sensor"}
  T21 = enum16{"Default", "Snail", "Random", "Snake", "Line"}
  T22 = enum32{"Microscope objective piezos", "Sample piezo stack"}
  T23 = cluster{"Scan Fast Axis":enum16{"Y", "X"}, "Scanning Mode":enum16{"Default", "Snail", "Random", "Snake", "Line"}, "Scan X Center (V)":dbl, "Scan X Res. (V)":dbl, "Scan X Tot. Length (V)":dbl, "Scan Y Center (V)":dbl, "Scan Y Res. (V)":dbl, "Scan Y Tot. Length":dbl}
  T24 = cluster{"Exposure Time (ms)":dbl, "Accumulations":dbl, "Excitation Wavelength (nm)":dbl, "Acq Mode":T3, "CCD ROI":enum16{"Custom ROI", "Full sensor", "Binned full sensor"}, "KCube Shutter On?":bool}
  T25 = enum32{"Spectrum", "XY Intensity Map", "Polar", "Contrast", "APDs", "PLE", "Conversions & info", "Settings", "Controls & indicators"}
  T26 = cluster{"Image":dbl[][][], "Frame Size":cluster{"F":i32, "Y":i32, "X":i32}}[]
  T27 = cluster{"LinT Start Pos (mm)":dbl, "LinT Step Pos (mm)":dbl, "LinT End pos (mm)":dbl, "LinTFine Start Pos (usteps)":dbl, "LinTFines Step Pos (usteps)":dbl, "LinTFine End Pos (usteps)":dbl}
  T28 = enum32{"Spectrum Acquisition", "Intensity Map Acquisition", "Polarisation Acquisition", "Contrast Acquisition", "APDs Acquisition", "Absorption", "Conversions", "Settings", "Controls & indicators"}
  T29 = enum8{"Enabled", "Disabled", "Disabled and Grayed Out"}
  T30 = enum16{"Contrast", "Spectre", "Polarisation", "Time Trace", "XY Intensity Map"}
  T31 = cluster{"Scan Main Progess Bar":refnum<vi>, "Acquire XY Map":refnum<vi>, "MasterPause":refnum<vi>, "MasterStop":refnum<vi>, "Save XY Map":refnum<vi>, "Scan X Readout (V)":refnum<vi>, "Scan Y Readout (V)":refnum<vi>, "CCD 1D Spectrum XY Map":refnum<vi>, "XY Intensity Map":refnum<vi>, "CCD 2D Image XY Map":refnum<vi>, "Expected (s)":refnum<vi>, "Elapsed (s)":refnum<vi>, "Cnts":refnum<vi>}
  T32 = cluster{"Acquire Polarisation":refnum<vi>, "Save Polarisation":refnum<vi>, "MasterPause":refnum<vi>, "MasterStop":refnum<vi>, "Scan Main Progess Bar":refnum<vi>, "RotStage Exc Angle Readout (°)":refnum<vi>, "RotStage Det Angle Readout (°)":refnum<vi>, "Polarisation 1D Spectrum":refnum<vi>, "Polarisation 2D Image":refnum<vi>, "Shutter Ctrls":refnum<vi>, "KCube Shutter Device Reference":refnum<vi>}
  T33 = typedef "LightField Automation.lvclass/OpticalPortLocation.ctl" = i32
  T34 = cluster{"Acq Time (ms)":dbl, "PLE Start (nm)":dbl, "PLE Step (nm)":dbl, "PLE End (nm)":dbl, "Spectrum Custom Mode":u16, "KCube Shutter On?":bool}
  T35 = cluster{"LightField Automation out":refnum<class "LightField Automation.lvclass">, "LightField error out":errorcluster, "VISA resource name out":refnum<visa-resource-name>, "ESP301 Error":errorcluster, "Photodiode handle out":refnum<visa-resource-name>, "Photodiode error out":errorcluster}
  T36 = cluster{"LightField Automation out":refnum<class "LightField Automation.lvclass">, "error out":errorcluster, "FSM X Task":refnum<k21>, "FSM Y Task":refnum<k21>}
  T37 = cluster{"LightField Automation out":refnum<class "LightField Automation.lvclass">, "error out":errorcluster, "Instrument Channel out":string, "error out":errorcluster, "ESP 301 COM out":refnum<visa-resource-name>, "ESP 301 error out":errorcluster, "Photodiode out":refnum<visa-resource-name>, "Photodiode error out":errorcluster}
  T38 = cluster{"PZA12 Positions":dbl[], "Contrast of ROI vs PZC":dbl[]}
  T39 = typedef "LVRangeTypeDef.ctl" = cluster{"Minimum":dbl, "Maximum":dbl, "Increment":dbl, "Minor Increment":dbl, "Start":dbl}
  T40 = cluster{"Sample first cooldown":timestamp, "SampleOf":string, "Synthesis/Name":string, "Synthesis/InjTemp":dbl, "Synthesis/Dilution":dbl, "Synthesis/Polymer":string, "Synthesis/DilutionPolyRatio":dbl, "Synthesis/Solvent":string}
  T41 = cluster{"Comment":string, "Temperature (K)":dbl, "Center Wavelength (nm)":dbl, dbl, "Excitation Source":enum16{"P", "CW", "SK"}, "Exposure Time (ms)":dbl, "Experiment Name With Date":string, "Acq Mode":T3, "Log file":string, "Exposure Time (ms)":dbl, "Wavelength calibration":dbl[], "Excitation Wavelength (nm)":dbl, "Grating":string, cluster{"Att Pos X":dbl, "Att Pos Y":dbl, "Att Pos Z":dbl, "Map Marker X Pos":i8, "Map Marker Y Pos":i8, "Scan X Readout (V)":dbl, "Scan Y Readout (V)":dbl}, cluster{"Sample first cooldown":timestamp, "SampleOf":string, "Synthesis/Name":string, "Synthesis/InjTemp":dbl, "Synthesis/Dilution":dbl, "Synthesis/Polymer":string, "Synthesis/DilutionPolyRatio":dbl, "Synthesis/Solvent":string}}
  T42 = enum16{"Time Trace", "Contrast", "XY Intensity Map", "Polarisation", "Spectrum", "Michelson", "fPow"}
  T43 = typedef "imagedata.ctl" = cluster{"image type":i32, "image depth":i32, "image":u8[], "mask":u8[], "colors":u32[], "Rectangle":cluster{"left":i16, "top":i16, "right":i16, "bottom":i16}}
  T44 = cluster{"Image":dbl[][][], "Frame Size":cluster{"F":i32, "Y":i32, "X":i32}}
  T45 = enum16{"Time Trace", "Contrast", "XY Intensity Map", "Polarisation", "Spectrum", "Michelson", "fPow", "PLE"}
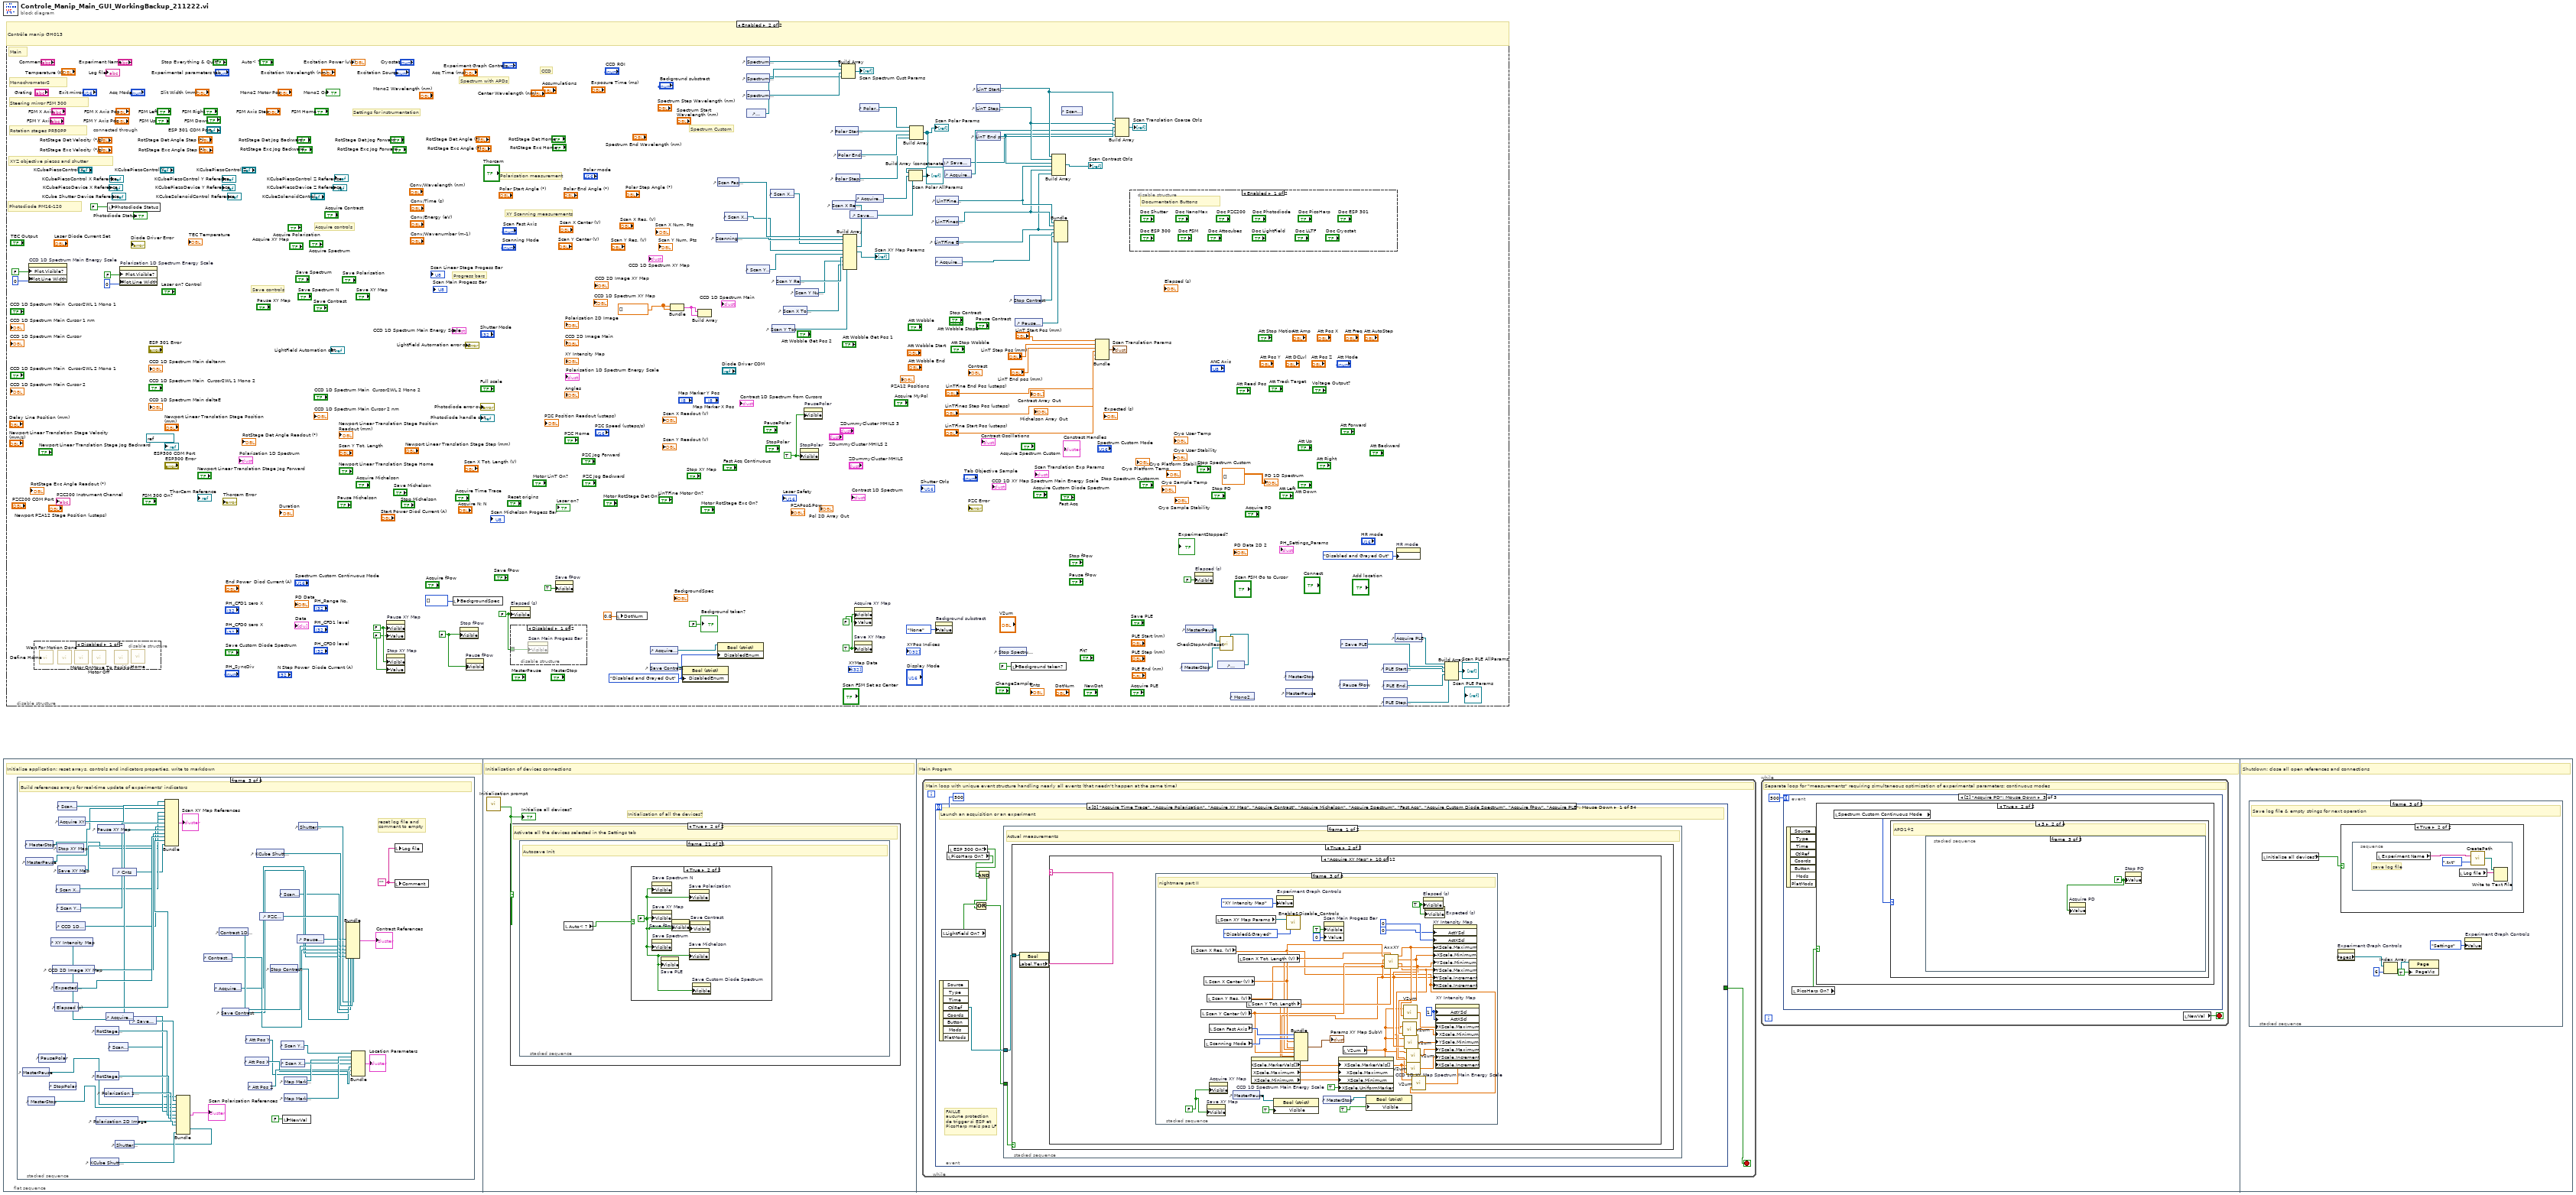
[diagram p0: block diagram]
diagram:
  n1 = flat-sequence {
    frame #0 {
      # "Initialise application: reset arrays, controls and indicators properties, write to markdown"
      n2 = stacked-sequence {
        frame #0 {
          # "Stop program if sample details are not all filled-in"
          n3 = local read "Write to Markdown?"() -> (w1:bool)
          n4 = case shown="False" w1 {
            frame True {
              n5 = local read "SampleGoal"() -> (w4:string)
              n6 = Equal?(x=w4, y="") -> (x = y?=w2:bool)
              n7 = case shown="True" w2 {
                frame False {
                }
                frame True {
                  n8 = call "Display Message to User"() -> ("OK"=w6:bool)  [unwired: 10 in, 1 out]
                  n9 = Stop(stop? (T)=w6) -> ()
                  n10 = property on="Experiment Graph Controls" class="TabCtl (strict)"("Value"=T25."Settings" ("Experiment Graph Controls")) -> ()  [unwired: 2 in, 2 out]
                }
              }
            }
            frame False {
              n11 = local read "SampleGoal"() -> (w9:string)
              n12 = Equal?(x=w9, y="") -> (x = y?=w7:bool)
              n13 = case shown="True" w7 {
                frame False {
                }
                frame True {
                  n14 = call "Display Message to User2"() -> ("OK"=w11:bool)  [unwired: 10 in, 1 out]
                  n15 = Not(x=w11) -> (.not. x?=w10:bool)
                  n16 = Stop(stop? (T)=w10) -> ()
                  n17 = property on="Experiment Graph Controls" class="TabCtl (strict)"("Value"=T25."Settings" ("Experiment Graph Controls")) -> ()  [unwired: 2 in, 2 out]
                }
              }
            }
          }
        }
        frame #1 {
          # "Write file header and sample details to Markdown"
          n18 = case shown="True" "Write to Markdown?" {
            frame False {
            }
            frame True {
              n19 = local read "Synthesis/DilutionPolyRatio"() -> (w26:dbl)
              n20 = local read "Sample first cooldown"() -> (w22:timestamp)
              n21 = local read "Synthesis/InjTemp"() -> (w29:dbl)
              n22 = local read "Synthesis/Polymer"() -> (w23:string)
              n23 = local read "Synthesis/Dilution"() -> (w27:dbl)
              n24 = local read "Synthesis/Solvent"() -> (w24:string)
              n25 = local read "Synthesis/Name"() -> (w28:string)
              n26 = local read "Synthesis/Name"() -> (w25:string)
              n27 = local read "SampleOf"() -> (w21:string)
              n28 = Bundle("Synthesis/InjTemp"=w29, "Synthesis/Name"=w28, "Synthesis/Dilution"=w27, "Synthesis/DilutionPolyRatio"=w26, "Synthesis/Name"=w25, "Synthesis/Solvent"=w24, "Synthesis/Polymer"=w23, "Sample first cooldown"=w22, "SampleOf"=w21) -> (w20:T2)  [unwired: 1 in]
              "output cluster" <- w20
              n29 = local read "Write to Markdown?"() -> (w18:bool)
              n30 = call "SampleDetails.vi"("SampleDetailsClus"=w20, "SampleGoal"="SampleGoal", "Wrte to Obs"=w18, "NewSampleDetails?"=TRUE, "Header?"=TRUE) -> ("SampleNameNoDate"=w15:string, "SampleName"=→"Experiment Name With Date":string)
              n31 = local write "Experiment Name"(w15) -> ()
            }
          }
        }
        frame #2 {
          w76 = ""
          # "reset log file and \ncomment to empty"
          # "Build references arrays for real-time update of experiments' indicators"
          n32 = control-ref of="MasterPause"() -> (w33:refnum<vi>)
          n33 = control-ref of="MasterStop"() -> (w30:refnum<vi>)
          n34 = control-ref of="MasterPause"() -> (w31:refnum<vi>)
          n35 = control-ref of="MasterStop"() -> (w32:refnum<vi>)
          n36 = control-ref of="PausePolar"() -> ()  [unwired: 1 out]
          n37 = control-ref of="StopPolar"() -> ()  [unwired: 1 out]
          n38 = control-ref of="XY Intensity Map"() -> (w51:refnum<vi>)
          n39 = control-ref of="CCD 2D Image XY Map"() -> (w52:refnum<vi>)
          n40 = control-ref of="Expected (s)"() -> (w53:refnum<vi>)
          n41 = control-ref of="Elapsed (s)"() -> (w54:refnum<vi>)
          n42 = control-ref of="Scan X Readout (V)"() -> (w48:refnum<vi>)
          n43 = control-ref of="CCD 1D Spectrum XY Map"() -> (w50:refnum<vi>)
          n44 = control-ref of="Stop XY Map"() -> ()  [unwired: 1 out]
          n45 = control-ref of="Scan Y Readout (V)"() -> (w49:refnum<vi>)
          n46 = control-ref of="Scan Main Progess Bar"() -> (w45:refnum<vi>)
          n47 = control-ref of="Save XY Map"() -> (w47:refnum<vi>)
          n48 = control-ref of="Acquire XY Map"() -> (w46:refnum<vi>)
          n49 = control-ref of="KCube Shutter Device Reference"() -> (w63:refnum<vi>)
          n50 = control-ref of="RotStage Exc Angle Readout (°)"() -> (w58:refnum<vi>)
          n51 = control-ref of="RotStage Det Angle Readout (°)"() -> (w59:refnum<vi>)
          n52 = control-ref of="Polarisation 2D Image"() -> (w61:refnum<vi>)
          n53 = control-ref of="Pause XY Map"() -> ()  [unwired: 1 out]
          n54 = control-ref of="Polarisation 1D Spectrum"() -> (w60:refnum<vi>)
          n55 = control-ref of="Acquire Polarisation"() -> (w55:refnum<vi>)
          n56 = control-ref of="Scan Main Progess Bar"() -> (w57:refnum<vi>)
          n57 = control-ref of="Cnts"() -> (w43:refnum<vi>)